vi "HFRR ADV v040.vi"() -> ()   [LabVIEW 2025] (continued)
          }
        }
        n1328 = case shown="True" w1638 {
          selector: w1638 -> [_ w1646]
          frame False {
          }
          frame True {
            n1329 = Not(x=w1646) -> (.not. x?=w1644:bool)
            n1330 = local write "CAMERA ROI MAX TEMP"(w1644) -> ()
            n1331 = call "IMAGE ANALYSIS.vi"("Enum"=POST_ANALYSIS_ENUM."SHOW UI") -> ("error out"=w1643:errorcluster)  [unwired: 9 in, 1 out]
            n1332 = call "LIST FILE NAMES.vi"("error in (no error)"=w1643) -> ("filenames"=w1642:string[])  [unwired: 9 in, 1 out]
            n1333 = property on="Test File List :" class="CmbBox"("Strings[]"=w1642) -> ()  [unwired: 2 in, 2 out]
          }
        }
        n1334 = local write "CAMERA ROI MIN TEMP"(TRUE ("CAMERA ROI MIN TEMP")) -> ()
      }
      frame "Compare Files" {
        n1335 = local read "LIVE FEED MIN TEMP"() -> (w1652:bool)
        n1336 = local write "LIVE FEED MAX TEMP"(TRUE ("LIVE FEED MAX TEMP")) -> ()
        n1337 = local read "CAMERA ROI MIN TEMP"() -> (w1650:bool)
        n1338 = case shown="True" w1652 {
          selector: w1652 -> [_ w1659]
          frame False {
          }
          frame True {
            n1339 = Not(x=w1659) -> (.not. x?=w1658:bool)
            n1340 = local write "LIVE FEED MIN TEMP"(w1658) -> ()
            n1341 = call "CAMERA LIVE FEED FGV.vi"("Enum - Menu"=CAMERA_LIVE_FEED_ENUM."CAMERA MINIMIZE") -> ()  [unwired: 9 in, 2 out]
          }
        }
        n1342 = case shown="True" w1650 {
          selector: w1650 -> [_ w1656]
          frame False {
          }
          frame True {
            n1343 = Not(x=w1656) -> (.not. x?=w1655:bool)
            n1344 = local write "CAMERA ROI MIN TEMP"(w1655) -> ()
            n1345 = call "IMAGE ANALYSIS.vi"("Enum"=POST_ANALYSIS_ENUM."MINIMIZE UI") -> ()  [unwired: 9 in, 2 out]
          }
        }
        n1346 = local write "CAMERA ROI MAX TEMP"(TRUE ("CAMERA ROI MAX TEMP")) -> ()
      }
      frame "About" {
        n1347 = local read "LIVE FEED MIN TEMP"() -> (w1662:bool)
        n1348 = local write "LIVE FEED MAX TEMP"(TRUE ("LIVE FEED MAX TEMP")) -> ()
        n1349 = local read "CAMERA ROI MIN TEMP"() -> (w1661:bool)
        n1350 = case shown="True" w1662 {
          selector: w1662 -> [_ w1669]
          frame False {
          }
          frame True {
            n1351 = Not(x=w1669) -> (.not. x?=w1668:bool)
            n1352 = local write "LIVE FEED MIN TEMP"(w1668) -> ()
            n1353 = call "CAMERA LIVE FEED FGV.vi"("Enum - Menu"=CAMERA_LIVE_FEED_ENUM."CAMERA MINIMIZE") -> ()  [unwired: 9 in, 2 out]
          }
        }
        n1354 = case shown="True" w1661 {
          selector: w1661 -> [_ w1666]
          frame False {
          }
          frame True {
            n1355 = Not(x=w1666) -> (.not. x?=w1665:bool)
            n1356 = local write "CAMERA ROI MIN TEMP"(w1665) -> ()
            n1357 = call "IMAGE ANALYSIS.vi"("Enum"=POST_ANALYSIS_ENUM."MINIMIZE UI") -> ()  [unwired: 9 in, 2 out]
          }
        }
        n1358 = local write "CAMERA ROI MAX TEMP"(TRUE ("CAMERA ROI MIN TEMP")) -> ()
      }
      frame "Advance" {
        n1359 = local read "LIVE FEED MIN TEMP"() -> (w1672:bool)
        n1360 = local write "LIVE FEED MAX TEMP"(TRUE ("LIVE FEED MAX TEMP")) -> ()
        n1361 = local read "CAMERA ROI MIN TEMP"() -> (w1670:bool)
        n1362 = case shown="True" w1672 {
          selector: w1672 -> [_ w1679]
          frame False {
          }
          frame True {
            n1363 = Not(x=w1679) -> (.not. x?=w1678:bool)
            n1364 = local write "LIVE FEED MIN TEMP"(w1678) -> ()
            n1365 = call "CAMERA LIVE FEED FGV.vi"("Enum - Menu"=CAMERA_LIVE_FEED_ENUM."CAMERA MINIMIZE") -> ()  [unwired: 9 in, 2 out]
          }
        }
        n1366 = local write "CAMERA ROI MAX TEMP"(TRUE ("CAMERA ROI MAX TEMP")) -> ()
        n1367 = case shown="True" w1670 {
          selector: w1670 -> [_ w1676]
          frame False {
          }
          frame True {
            n1368 = Not(x=w1676) -> (.not. x?=w1675:bool)
            n1369 = local write "CAMERA ROI MIN TEMP"(w1675) -> ()
            n1370 = call "IMAGE ANALYSIS.vi"("Enum"=POST_ANALYSIS_ENUM."MINIMIZE UI") -> ()  [unwired: 9 in, 2 out]
          }
        }
      }
      frame "Mooha" {
        n1371 = local read "LIVE FEED MIN TEMP"() -> (w1682:bool)
        n1372 = local write "LIVE FEED MAX TEMP"(TRUE ("LIVE FEED MAX TEMP")) -> ()
        n1373 = local read "CAMERA ROI MIN TEMP"() -> (w1680:bool)
        n1374 = case shown="True" w1682 {
          selector: w1682 -> [_ w1689]
          frame False {
          }
          frame True {
            n1375 = Not(x=w1689) -> (.not. x?=w1688:bool)
            n1376 = local write "LIVE FEED MIN TEMP"(w1688) -> ()
            n1377 = call "CAMERA LIVE FEED FGV.vi"("Enum - Menu"=CAMERA_LIVE_FEED_ENUM."CAMERA MINIMIZE") -> ()  [unwired: 9 in, 2 out]
          }
        }
        n1378 = local write "CAMERA ROI MAX TEMP"(TRUE ("CAMERA ROI MAX TEMP")) -> ()
        n1379 = case shown="True" w1680 {
          selector: w1680 -> [_ w1686]
          frame False {
          }
          frame True {
            n1380 = Not(x=w1686) -> (.not. x?=w1685:bool)
            n1381 = local write "CAMERA ROI MIN TEMP"(w1685) -> ()
            n1382 = call "IMAGE ANALYSIS.vi"("Enum"=POST_ANALYSIS_ENUM."MINIMIZE UI") -> ()  [unwired: 9 in, 2 out]
          }
        }
      }
    }
    n1383 = local read "Auto Start Test"() -> (w1427:bool)
    n1384 = case shown="True" "sign in temp" {
      frame False {
      }
      frame True {
        w1462 = 1 ("y")
        n1385 = local read "USERNAME"() -> (w1468:string)
        n1386 = local read "USER ID"() -> (w1465:string)
        n1387 = call <vilib>:"Trim Whitespace.vi"("string"=w1468) -> ("trimmed string"=w1467:string)  [unwired: 1 in]
        n1388 = call <vilib>:"Trim Whitespace.vi"("string"=w1465) -> ("trimmed string"=w1466:string)  [unwired: 1 in]
        n1389 = String Length(string=w1467) -> (length=w1464:i32)
        n1390 = String Length(string=w1466) -> (length=w1463:i32)
        n1391 = Greater?(x=w1464, y=w1462) -> (0:w1461:bool)
        n1392 = Greater?(x=w1463, y=w1462) -> (0:w1460:bool)
        n1393 = And(x=w1461, y=w1460) -> (x .and. y?=w1459:bool)
        n1394 = case shown="True" w1459 {
          frame False {
            n1395 = property on="Sign In" class="Bool (strict)"("DisabledEnum"=T19."Disabled" ("Disabled")) -> ()  [unwired: 2 in, 2 out]
          }
          frame True {
            n1396 = property on="Sign In" class="Bool (strict)"("DisabledEnum"=T19."Enabled" ("Disabled")) -> ()  [unwired: 2 in, 2 out]
          }
        }
      }
    }
    n1397 = local read "Air Temperature"() -> (w1444:bool)
    n1398 = local read "Coefficient Of Friction"() -> (w1445:bool)
    n1399 = case shown="False" w1427 {
      frame False {
        n1400 = local read "Auto stop temp"() -> (w1456:bool)
        n1401 = case shown="True" w1456 {
          frame False {
          }
          frame True {
            n1402 = local write "Auto Start Temp"(FALSE ("Auto Start Temp")) -> ()
          }
        }
      }
      frame True {
        "Auto stop temp" <- TRUE ("Auto stop temp")
      }
    }
    n1403 = local read "Humidity"() -> (w1443:bool)
    n1404 = case shown="\"HOME\"" w1453 {
      frame "HOME" {
        n1405 = local write "main tab sub"(enum32{"Page 1", "Page 2"}."Page 1" ("main tab sub")) -> ()
      }
      frame Default {
        n1406 = local write "main tab sub"(enum32{"Page 1", "Page 2"}."Page 2" ("main tab sub")) -> ()
      }
    }
    n1407 = case shown="True" w1452 {
      selector: w1452 -> [_ w1804]
      frame False {
      }
      frame True {
        n1408 = Not(x=w1804) -> (.not. x?=w1803:bool)
        n1409 = local write "Sign In"(w1803) -> ()
        n1410 = local write "Main Dashboard Buttons"(T26."Test Setup" ("Main Dashboard Buttons")) -> ()
      }
    }
    n1411 = case shown="\"Numeric Display\", Default" "Num/Graph" {
      frame "Numeric Display", Default {
        n1412 = property on="Single/Multiple" class="RadioBtnsControl (strict)"("Visible"=FALSE) -> ()  [unwired: 2 in, 2 out]
        n1413 = property on="Single - Graph" class="Ring (strict)"("Visible"=FALSE) -> ()  [unwired: 2 in, 2 out]
        n1414 = local write "Main Tab Display"(T4."Dashboard 1" ("Main Tab Display")) -> ()
      }
      frame "Graph Display" {
        n1415 = property on="Single/Multiple" class="RadioBtnsControl (strict)"("Visible"=TRUE) -> ()  [unwired: 2 in, 2 out]
        n1416 = case shown="\"Multiple\"" "Single/Multiple" {
          frame "Single ", Default {
            n1417 = property on="Single - Graph" class="Ring (strict)"("Visible"=TRUE) -> ()  [unwired: 2 in, 2 out]
            n1418 = local write "Main Tab Display"(T4."Dashboard 3" ("Main Tab Display")) -> ()
          }
          frame "Multiple" {
            n1419 = property on="Single - Graph" class="Ring (strict)"("Visible"=FALSE) -> ()  [unwired: 2 in, 2 out]
            n1420 = local write "Main Tab Display"(T4."Dashboard 2" ("Main Tab Display")) -> ()
          }
        }
      }
    }
    n1421 = local read "Stroke"() -> (w1442:bool)
    n1422 = local read "USERNAME"() -> (w1447:string)
    n1423 = case shown="True" w1445 {
      selector: w1445 -> [_ w1729]
      frame False {
      }
      frame True {
        n1424 = Not(x=w1729) -> (.not. x?=w1728:bool)
        n1425 = local write "Coefficient Of Friction"(w1728) -> ()
        n1426 = local write "Tab Control 2"(T6."Coefficient Of Friction" ("Tab Control 2")) -> ()
      }
    }
    n1427 = case shown="True" w1444 {
      selector: w1444 -> [_ w1726]
      frame False {
      }
      frame True {
        n1428 = Not(x=w1726) -> (.not. x?=w1724:bool)
        n1429 = local write "Air Temperature"(w1724) -> ()
        n1430 = local write "Tab Control 2"(T6."Air Temperature" ("Tab Control 2")) -> ()
      }
    }
    n1431 = case shown="True" w1442 {
      selector: w1442 -> [_ w1720]
      frame False {
      }
      frame True {
        n1432 = Not(x=w1720) -> (.not. x?=w1718:bool)
        n1433 = local write "Stroke"(w1718) -> ()
        n1434 = local write "Tab Control 2"(T6."Stroke" ("Tab Control 2")) -> ()
      }
    }
    n1435 = local write "tested by"(w1447) -> ()
    n1436 = case shown="True" w1443 {
      selector: w1443 -> [_ w1723]
      frame False {
      }
      frame True {
        n1437 = Not(x=w1723) -> (.not. x?=w1721:bool)
        n1438 = local write "Humidity"(w1721) -> ()
        n1439 = local write "Tab Control 2"(T6."Humidity" ("Tab Control 2")) -> ()
      }
    }
    n1440 = case shown="\"Calibration\"" "Main Dashboard Buttons" {
      tunnel: [T2."HOME" ("Main Tab") T2."Test Setup" ("Main Tab") T2."Acquire" ("Main Tab") T2."Adv Scar" ("Main Tab") T2."Adv Scar Report" ("Main Tab") T2."Compare Files" ("Main Tab") T2."Calibration" ("Main Tab") T2."About" ("Main Tab") T2."Advance" ("Main Tab")] -> w1426
      frame "Home", Default {
      }
      frame "Test Setup" {
      }
      frame "Dashboard" {
      }
      frame "Imaging" {
      }
      frame "Report" {
      }
      frame "Analysis" {
      }
      frame "Calibration" {
      }
      frame "About" {
      }
      frame "Advance" {
      }
    }
    n1441 = Wait (ms)(milliseconds to wait=u32 100) -> ()  [unwired: 1 out]
    n1442 = local read "Main Tab Display"() -> (w1446:T4)
    n1443 = local write "Main Tab"(w1426) -> ()
    n1444 = case shown="\"Dashboard 3\"" w1446 {
      frame "Dashboard 1", Default {
        n1445 = property on="Reset Graph" class="Bool (strict)"("Visible"=FALSE) -> ()  [unwired: 2 in, 2 out]
      }
      frame "Dashboard 2" {
        n1446 = property on="Reset Graph" class="Bool (strict)"("Visible"=TRUE) -> ()  [unwired: 2 in, 2 out]
      }
      frame "Dashboard 3" {
        n1447 = property on="Reset Graph" class="Bool (strict)"("Visible"=TRUE) -> ()  [unwired: 2 in, 2 out]
      }
    }
    n1448 = local read "SCAR MEASURMENT"() -> (w1434:enum32{"Auto Scar", "Manual Scar"})
    n1449 = local read "Humidity"() -> (w1448:bool)
    n1450 = local read "Cap Live Image"() -> (w1431:bool)
    n1451 = local read "Sample Temperature"() -> (w1441:bool)
    n1452 = local read "Air Temp vs Humidity"() -> (w1439:bool)
    n1453 = local read "Frequency"() -> (w1440:bool)
    n1454 = case shown="False" w1448 {
      frame False {
        n1455 = local write "Humidity On Command"(TRUE ("Humidity On Command")) -> ()
        n1456 = case shown="True" "Humidity Off Command" {
          selector: "Humidity Off Command" -> [_ w1736]
          frame False {
          }
          frame True {
            n1457 = stacked-sequence {
              frame #0 {
                n1458 = local read "WriteHumidity"() -> (w1738:string[])
                n1459 = Insert Into Array(array=w1738, new element="R;1" ("new element/subarray")) -> (w1737:string[])  [unwired: 1 in]
                n1460 = local write "WriteHumidity"(w1737) -> ()
              }
              frame #1 {
                n1461 = Wait (ms)(milliseconds to wait=u32 500) -> ()  [unwired: 1 out]
              }
              frame #2 {
                n1462 = local read "WriteHumidity"() -> (w1742:string[])
                n1463 = local read "EVENT LOG"() -> (w1746:string)
                n1464 = call "Event Log.vi"("Content"="Humidity Control Off" ("string"), "EVENT LOG"=w1746) -> ("EVENT LOG"=w1747:string)  [unwired: 8 in, 1 out]
                n1465 = local write "EVENT LOG"(w1747) -> ()
                n1466 = Insert Into Array(array=w1742, new element="R;1" ("new element/subarray")) -> (w1743:string[])  [unwired: 1 in]
                n1467 = local write "WriteHumidity"(w1743) -> ()
                n1468 = local write "Humidity 2"(TRUE ("Humidity")) -> ()
              }
            }
            n1469 = Not(x=w1736) -> (.not. x?=w1735:bool)
            n1470 = local write "Humidity Off Command"(w1735) -> ()
          }
        }
      }
      frame True {
        n1471 = local write "Humidity Off Command"(TRUE ("Humidity Off Command")) -> ()
        n1472 = case shown="False" "Humidity On Command" {
          selector: "Humidity On Command" -> [_ w1751]
          frame False {
          }
          frame True {
            n1473 = stacked-sequence {
              frame #0 {
                n1474 = local read "Set Rh"() -> (w1757:dbl)
                n1475 = local read "WriteHumidity"() -> (w1753:string[])
                n1476 = Number To Fractional String(number=w1757, precision (6)=i16 2) -> (F-format string=w1758:string)  [unwired: 2 in]
                n1477 = Concatenate Strings("M;" ("new element/subarray"), w1758) -> (w1756:string)
                n1478 = Insert Into Array(array=w1753, new element=w1756) -> (w1752:string[])  [unwired: 1 in]
                n1479 = local write "WriteHumidity"(w1752) -> ()
              }
              frame #1 {
                n1480 = Wait (ms)(milliseconds to wait=u32 500) -> ()  [unwired: 1 out]
              }
              frame #2 {
                n1481 = local read "WriteHumidity"() -> (w1761:string[])
                n1482 = local read "Set Rh"() -> (w1765:dbl)
                n1483 = Number To Fractional String(number=w1765, precision (6)=i16 2) -> (F-format string=w1766:string)  [unwired: 2 in]
                n1484 = Concatenate Strings("M;" ("new element/subarray"), w1766) -> (w1764:string)
                n1485 = Insert Into Array(array=w1761, new element=w1764) -> (w1760:string[])  [unwired: 1 in]
                n1486 = local write "WriteHumidity"(w1760) -> ()
              }
              frame #3 {
                n1487 = Wait (ms)(milliseconds to wait=u32 500) -> ()  [unwired: 1 out]
              }
              frame #4 {
                (unwired) "% RH" ("string")
                (unwired) i16 2 ("precision (6)")
                (unwired) "M;" ("new element/subarray")
                n1488 = local read "Set Rh"() -> (w1775:dbl)
                n1489 = local read "WriteHumidity"() -> (w1768:string[])
                n1490 = Number To Fractional String(number=w1775, precision (6)=i16 2) -> (F-format string=w1772:string)  [unwired: 2 in]
                n1491 = Concatenate Strings("M;" ("new element/subarray"), w1772) -> (w1776:string)
                n1492 = Concatenate Strings("Humidity Set to : " ("string"), w1772, "% RH" ("string")) -> (w1770:string)
                n1493 = Insert Into Array(array=w1768, new element=w1776) -> (w1769:string[])  [unwired: 1 in]
                n1494 = disable-structure shown="Enabled" {
                  frame Enabled {
                    n1495 = local read "EVENT LOG"() -> (w1779:string)
                    n1496 = call "Event Log.vi"("Content"="Humidity Control On", "EVENT LOG"=w1779) -> ("EVENT LOG"=w1780:string)  [unwired: 8 in, 1 out]
                    n1497 = local write "EVENT LOG"(w1780) -> ()
                  }
                  frame Disabled {
                  }
                }
                n1498 = disable-structure shown="Enabled" {
                  disable-tunnel: w1770 -> [_ _]
                  frame Enabled {
                    n1499 = local read "EVENT LOG"() -> (w1782:string)
                    n1500 = call "Event Log.vi"("Content"="Humidity Control On", "EVENT LOG"=w1782) -> ("EVENT LOG"=w1783:string)  [unwired: 8 in, 1 out]
                    n1501 = local write "EVENT LOG"(w1783) -> ()
                  }
                  frame Disabled {
                  }
                }
                n1502 = local write "WriteHumidity"(w1769) -> ()
              }
            }
            n1503 = Not(x=w1751) -> (.not. x?=w1750:bool)
            n1504 = local write "Humidity On Command"(w1750) -> ()
          }
        }
      }
    }
    n1505 = Equal?(x=w1434, y=enum32{"Auto Scar", "Manual Scar"}."Auto Scar" ("SCAR MEASURMENT")) -> (x = y?=w1430:bool)
    n1506 = local read "TEST STANDARD"() -> (w1437:T3)
    n1507 = And(x=w1431, y=w1430) -> (x .and. y?=w1432:bool)
    n1508 = case shown="True" w1432 {
      selector: w1432 -> [_ w1535]
      tunnel: errorcluster {"status"=FALSE, "code"=0, "source"=""} ("error in (no error) 3") -> [_ w1536]
      frame False {
      }
      frame True {
        n1509 = stacked-sequence {
          tunnel: w1536 -> [_ _ _ _ _ _ _ w1584]
          tunnel: w1535 -> [_ _ _ _ _ w1565 _ _]
          frame #0 {
            n1510 = call "CAMERA LIVE FEED FGV.vi"("Enum - Menu"=CAMERA_LIVE_FEED_ENUM."CAMERA MINIMIZE") -> ()  [unwired: 9 in, 2 out]
          }
          frame #1 {
            n1511 = property on="Auto Scar Check  2" class="Clust (strict)"("Visible"=TRUE) -> ()  [unwired: 2 in, 2 out]
          }
          frame #2 {
            n1512 = String To Path(string="C:\\LAB-IQ\\Image Calibrate v01.dcf") -> (path=w1541:path)
            n1513 = Open/Create/Replace File ("Open File")(file path (use dialog)=w1541) -> (refnum out=w1542:refnum<file>)  [unwired: 5 in, 2 out]
            n1514 = for {
              N: 4 -> [_]
              tunnel: w1542 -> [w1548]
              i -> [w1544]
              n1515 = Read from Text File ("Read File")(file (use dialog)=w1548) -> (text=w1549:string)  [unwired: 3 in, 3 out]
              n1516 = String Subset(string=w1549, offset (0)=6, length (rest)=10 ("length (rest)")) -> (substring=w1545:string)
              n1517 = Fract/Exp String To Number(string=w1545) -> (number=w1543:dbl)  [unwired: 3 in, 1 out]
              n1518 = case shown="0" w1544 {
                tunnel: w1543 -> [w1550 w1551 _ w1552 _]
                frame 0 {
                  "5x Gain" <- w1550
                }
                frame 1 {
                  "10x Gain" <- w1551
                }
                frame 2 {
                }
                frame 3 {
                  "100x gain" <- w1552
                }
                frame 4, Default {
                }
              }
            }
          }
          frame #3 {
            n1519 = local read "FILE 3"() -> (w1558:string)
            n1520 = call <vilib>:"Trim Whitespace.vi"("string"="C:\\LAB-IQ\\images\\") -> ("trimmed string"=w1560:string)  [unwired: 1 in]
            n1521 = String To Path(string=w1560) -> (path=w1559:path)
            n1522 = Concatenate Strings(w1558, ".png" ("string")) -> (w1557:string)
            n1523 = Build Path(base path=w1559, name or relative path=w1557) -> (appended path=w1555:path)
            "Image path" <- w1555
            n1524 = Path To String(path=w1555) -> (string=w1554:string)
            n1525 = call "CAMERA LIVE FEED FGV.vi"("Enum - Menu"=CAMERA_LIVE_FEED_ENUM."CAMERA SAVE", "Image Path"=w1554) -> ()  [unwired: 8 in, 2 out]
          }
          frame #4 {
            n1526 = One Button Dialog(message="Image saved successfully") -> ()  [unwired: 1 in, 1 out]
          }
          frame #5 {
            n1527 = local read "TEST STANDARD"() -> (w1564:T3)
            n1528 = local read "Magnification len live scar"() -> (w1576:string)
            n1529 = Not(x=w1565) -> (.not. x?=w1566:bool)
            n1530 = local write "Cap Live Image"(w1566) -> ()
            n1531 = case shown="\"ISO 12156\"" w1564 {
              tunnel: ["ASTM D6079" "ISO 12156"] -> w1563
              frame "ASTM D6079", Default {
              }
              frame "ISO 12156" {
              }
            }
            n1532 = case shown="\"5x\", Default" w1576 {
              tunnel: [w1579 w1580] -> w1575
              frame "5x", Default {
                n1533 = local read "5x Gain"() -> (w1579:dbl)
              }
              frame "10x" {
                # "5x"
                n1534 = local read "10x Gain"() -> (w1580:dbl)
              }
            }
            n1535 = local read "Image path"() -> (w1574:path)
            n1536 = local read "FILE 3"() -> (w1567:string)
            n1537 = call "EDGE DETCTION.vi"("GAIN VALUE"=w1575, "Image Path"=w1574) -> ("error out"=w1573:errorcluster, "return value"=w1572:cluster{string, string, dbl, dbl, dbl})  [unwired: 8 in]
            n1538 = Bundle By Name(cluster=T27 {"File Name"="", "Test Method"="", "Operator"="", "Fuel Description"="", "Date and time"=""} ("Main Ref"), "File Name"=w1567, "Test Method"=w1563) -> (w1568:T27)
            n1539 = call "duf file read.vi"("error in (no error)"=w1573, "Main Ref"=w1568) -> ("error out"=w1571:errorcluster, "Main Ref 2"=w1569:T27)  [unwired: 8 in]
            n1540 = call "EDGE DETECTION REPORT.vi"("error in (no error)"=w1571, "return value 2"=w1572, "Main Ref"=w1569) -> ()  [unwired: 8 in, 1 out]
          }
          frame #6 {
            n1541 = property on="Auto Scar Check  2" class="Clust (strict)"("Visible"=FALSE) -> ()  [unwired: 2 in, 2 out]
          }
          frame #7 {
            n1542 = call "CAMERA LIVE FEED FGV.vi"("Enum - Menu"=CAMERA_LIVE_FEED_ENUM."CAMERA MINIMIZE", "error in (no error)"=w1584) -> ()  [unwired: 8 in, 2 out]
            n1543 = local write "Main Dashboard Buttons"(T1."Home" ("Main Dashboard Buttons")) -> ()
            n1544 = local write "Main Tab"(T2."HOME" ("Main Tab")) -> ()
          }
        }
      }
    }
    n1545 = local read "Heater Button"() -> (w1438:bool)
    n1546 = case shown="True" w1440 {
      selector: w1440 -> [_ w1714]
      frame False {
      }
      frame True {
        n1547 = Not(x=w1714) -> (.not. x?=w1712:bool)
        n1548 = local write "Frequency"(w1712) -> ()
        n1549 = local write "Tab Control 2"(T6."Frequency" ("Tab Control 2")) -> ()
      }
    }
    n1550 = case shown="True" w1439 {
      selector: w1439 -> [_ w1711]
      frame False {
      }
      frame True {
        n1551 = Not(x=w1711) -> (.not. x?=w1709:bool)
        n1552 = local write "Air Temp vs Humidity"(w1709) -> ()
        n1553 = local write "Tab Control 2"(T6."Air Temp vs Rh" ("Tab Control 2")) -> ()
      }
    }
    n1554 = case shown="True" w1441 {
      selector: w1441 -> [_ w1717]
      frame False {
      }
      frame True {
        n1555 = Not(x=w1717) -> (.not. x?=w1715:bool)
        n1556 = local write "Sample Temperature"(w1715) -> ()
        n1557 = local write "Tab Control 2"(T6."Sample Temperature" ("Tab Control 2")) -> ()
      }
    }
    n1558 = case shown="\"Custom\"" w1437 {
      frame "ASTM D6079", Default {
        w1690 = "ASTM D6079 TEST CONDITIONS" ("Standard 2")
        n1559 = local write "Standard 2"(w1690) -> ()
        n1560 = local write "Standard"(w1690) -> ()
      }
      frame "ISO 12156" {
        w1691 = "ISO 12156 TEST CONDITIONS" ("Standard 2")
        n1561 = local write "Standard 2"(w1691) -> ()
        n1562 = local write "Standard"(w1691) -> ()
      }
      frame "CEC F-096-A-06" {
        w1692 = "CEC F-096-A-06 TEST CONDITIONS" ("Standard 2")
        n1563 = local write "Standard 2"(w1692) -> ()
        n1564 = local write "Standard"(w1692) -> ()
      }
      frame "Custom" {
        w1693 = "CUSTOM TEST CONDITIONS" ("Standard 2")
        n1565 = local write "Standard 2"(w1693) -> ()
        n1566 = local write "Standard"(w1693) -> ()
      }
    }
    n1567 = case shown="True" w1438 {
      frame False {
        n1568 = local write "Temperature On Command"(TRUE ("Temperature On Command")) -> ()
        n1569 = case shown="True" "Temperature Off Command" {
          selector: "Temperature Off Command" -> [_ w1697]
          frame False {
          }
          frame True {
            n1570 = Not(x=w1697) -> (.not. x?=w1696:bool)
            n1571 = local read "EVENT LOG"() -> (w1700:string)
            n1572 = local write "Temperature Off Command"(w1696) -> ()
            n1573 = call "Event Log.vi"("Content"="Heater Off", "EVENT LOG"=w1700) -> ("EVENT LOG"=w1699:string)  [unwired: 8 in, 1 out]
            n1574 = local write "EVENT LOG"(w1699) -> ()
          }
        }
      }
      frame True {
        n1575 = local write "Temperature Off Command"(TRUE ("Temperature Off Command")) -> ()
        n1576 = case shown="True" "Temperature On Command" {
          selector: "Temperature On Command" -> [_ w1704]
          frame False {
          }
          frame True {
            n1577 = Not(x=w1704) -> (.not. x?=w1703:bool)
            n1578 = local write "Temperature On Command"(w1703) -> ()
            n1579 = disable-structure shown="Enabled" {
              disable-tunnel: "Heater On" -> [w1706 _]
              frame Enabled {
                n1580 = local read "EVENT LOG"() -> (w1707:string)
                n1581 = call "Event Log.vi"("Content"=w1706, "EVENT LOG"=w1707) -> ("EVENT LOG"=w1708:string)  [unwired: 8 in, 1 out]
                n1582 = local write "EVENT LOG"(w1708) -> ()
              }
              frame Disabled {
              }
            }
          }
        }
      }
    }
    n1583 = local read "Main Tab"() -> (w1429:T2)
    n1584 = case shown="\"About\"" w1429 {
      frame "HOME", Default {
        w1471 = T19."Enabled" ("Disabled")
        n1585 = local read "Service Password enable"() -> (w1473:bool)
        n1586 = property on="Imaging" class="Bool (strict)"("DisabledEnum"=w1471) -> ()  [unwired: 2 in, 2 out]
        n1587 = property on="Dashboard" class="Bool (strict)"("DisabledEnum"=w1471) -> ()  [unwired: 2 in, 2 out]
        n1588 = property on="Test Setup" class="Bool (strict)"("DisabledEnum"=w1471) -> ()  [unwired: 2 in, 2 out]
        n1589 = property on="Analysis" class="Bool (strict)"("DisabledEnum"=w1471) -> ()  [unwired: 2 in, 2 out]
        n1590 = property on="Home" class="Bool (strict)"("DisabledEnum"=w1471) -> ()  [unwired: 2 in, 2 out]
        n1591 = property on="Report" class="Bool (strict)"("DisabledEnum"=w1471) -> ()  [unwired: 2 in, 2 out]
        n1592 = property on="Main Dashboard Buttons" class="RadioBtnsControl (strict)"("DisabledEnum"=w1471) -> ()  [unwired: 2 in, 2 out]
        n1593 = property on="Calibration" class="Bool (strict)"("DisabledEnum"=w1471) -> ()  [unwired: 2 in, 2 out]
        n1594 = case shown="True" w1473 {
          tunnel: [T19."Disabled" ("Disabled") T19."Enabled" ("Disabled")] -> w1472
          frame False {
          }
          frame True {
          }
        }
        n1595 = property on="About" class="Bool (strict)"("DisabledEnum"=w1472) -> ()  [unwired: 2 in, 2 out]
      }
      frame "Test Setup" {
        w1478 = T19."Enabled" ("Disabled")
        n1596 = local read "Service Password enable"() -> (w1477:bool)
        n1597 = property on="Dashboard" class="Bool (strict)"("DisabledEnum"=T19."Disabled" ("Disabled")) -> ()  [unwired: 2 in, 2 out]
        n1598 = property on="Imaging" class="Bool (strict)"("DisabledEnum"=w1478) -> ()  [unwired: 2 in, 2 out]
        n1599 = property on="Analysis" class="Bool (strict)"("DisabledEnum"=w1478) -> ()  [unwired: 2 in, 2 out]
        n1600 = property on="Home" class="Bool (strict)"("DisabledEnum"=w1478) -> ()  [unwired: 2 in, 2 out]
        n1601 = property on="Report" class="Bool (strict)"("DisabledEnum"=w1478) -> ()  [unwired: 2 in, 2 out]
        n1602 = property on="Test Setup" class="Bool (strict)"("DisabledEnum"=w1478) -> ()  [unwired: 2 in, 2 out]
        n1603 = case shown="True" w1477 {
          tunnel: [T19."Disabled" ("Disabled") T19."Enabled" ("Disabled")] -> w1476
          frame False {
          }
          frame True {
          }
        }
        n1604 = property on="About" class="Bool (strict)"("DisabledEnum"=w1476) -> ()  [unwired: 2 in, 2 out]
      }
      frame "Adv Scar" {
        w1485 = T19."Enabled" ("Disabled")
        n1605 = property on="Dashboard" class="Bool (strict)"("DisabledEnum"=T19."Disabled" ("Disabled")) -> ()  [unwired: 2 in, 2 out]
        n1606 = property on="Imaging" class="Bool (strict)"("DisabledEnum"=w1485) -> ()  [unwired: 2 in, 2 out]
        n1607 = property on="Analysis" class="Bool (strict)"("DisabledEnum"=w1485) -> ()  [unwired: 2 in, 2 out]
        n1608 = property on="Home" class="Bool (strict)"("DisabledEnum"=w1485) -> ()  [unwired: 2 in, 2 out]
        n1609 = property on="Report" class="Bool (strict)"("DisabledEnum"=w1485) -> ()  [unwired: 2 in, 2 out]
        n1610 = property on="Test Setup" class="Bool (strict)"("DisabledEnum"=w1485) -> ()  [unwired: 2 in, 2 out]
        n1611 = local read "Service Password enable"() -> (w1483:bool)
        n1612 = case shown="True" w1483 {
          tunnel: [T19."Disabled" ("Disabled") T19."Enabled" ("Disabled")] -> w1482
          frame False {
          }
          frame True {
          }
        }
        n1613 = property on="About" class="Bool (strict)"("DisabledEnum"=w1482) -> ()  [unwired: 2 in, 2 out]
      }
      frame "Calibration" {
        w1488 = T19."Enabled" ("Disabled")
        n1614 = property on="Dashboard" class="Bool (strict)"("DisabledEnum"=T19."Disabled" ("Disabled")) -> ()  [unwired: 2 in, 2 out]
        n1615 = property on="Imaging" class="Bool (strict)"("DisabledEnum"=w1488) -> ()  [unwired: 2 in, 2 out]
        n1616 = property on="Analysis" class="Bool (strict)"("DisabledEnum"=w1488) -> ()  [unwired: 2 in, 2 out]
        n1617 = property on="Home" class="Bool (strict)"("DisabledEnum"=w1488) -> ()  [unwired: 2 in, 2 out]
        n1618 = property on="Report" class="Bool (strict)"("DisabledEnum"=w1488) -> ()  [unwired: 2 in, 2 out]
        n1619 = property on="Test Setup" class="Bool (strict)"("DisabledEnum"=w1488) -> ()  [unwired: 2 in, 2 out]
        n1620 = local read "Service Password enable"() -> (w1490:bool)
        n1621 = property on="Calibration" class="Bool (strict)"("DisabledEnum"=w1488) -> ()  [unwired: 2 in, 2 out]
        n1622 = case shown="True" w1490 {
          tunnel: [T19."Disabled" ("Disabled") T19."Enabled" ("Disabled")] -> w1489
          frame False {
          }
          frame True {
          }
        }
        n1623 = property on="About" class="Bool (strict)"("DisabledEnum"=w1489) -> ()  [unwired: 2 in, 2 out]
      }
      frame "Adv Scar Report" {
        w1496 = T19."Enabled" ("Disabled")
        n1624 = property on="Dashboard" class="Bool (strict)"("DisabledEnum"=T19."Disabled" ("Disabled")) -> ()  [unwired: 2 in, 2 out]
        n1625 = property on="Imaging" class="Bool (strict)"("DisabledEnum"=w1496) -> ()  [unwired: 2 in, 2 out]
        n1626 = property on="Analysis" class="Bool (strict)"("DisabledEnum"=w1496) -> ()  [unwired: 2 in, 2 out]
        n1627 = property on="Home" class="Bool (strict)"("DisabledEnum"=w1496) -> ()  [unwired: 2 in, 2 out]
        n1628 = property on="Report" class="Bool (strict)"("DisabledEnum"=w1496) -> ()  [unwired: 2 in, 2 out]
        n1629 = property on="Test Setup" class="Bool (strict)"("DisabledEnum"=w1496) -> ()  [unwired: 2 in, 2 out]
        n1630 = local read "Service Password enable"() -> (w1495:bool)
        n1631 = case shown="True" w1495 {
          tunnel: [T19."Disabled" ("Disabled") T19."Enabled" ("Disabled")] -> w1494
          frame False {
          }
          frame True {
          }
        }
        n1632 = property on="About" class="Bool (strict)"("DisabledEnum"=w1494) -> ()  [unwired: 2 in, 2 out]
      }
      frame "Compare Files" {
        w1502 = T19."Enabled" ("Disabled")
        n1633 = local read "Service Password enable"() -> (w1501:bool)
        n1634 = property on="Dashboard" class="Bool (strict)"("DisabledEnum"=T19."Disabled" ("Disabled")) -> ()  [unwired: 2 in, 2 out]
        n1635 = property on="Imaging" class="Bool (strict)"("DisabledEnum"=w1502) -> ()  [unwired: 2 in, 2 out]
        n1636 = property on="Analysis" class="Bool (strict)"("DisabledEnum"=w1502) -> ()  [unwired: 2 in, 2 out]
        n1637 = property on="Home" class="Bool (strict)"("DisabledEnum"=w1502) -> ()  [unwired: 2 in, 2 out]
        n1638 = property on="Report" class="Bool (strict)"("DisabledEnum"=w1502) -> ()  [unwired: 2 in, 2 out]
        n1639 = property on="Test Setup" class="Bool (strict)"("DisabledEnum"=w1502) -> ()  [unwired: 2 in, 2 out]
        n1640 = case shown="True" w1501 {
          tunnel: [T19."Disabled" ("Disabled") T19."Enabled" ("Disabled")] -> w1500
          frame False {
          }
          frame True {
          }
        }
        n1641 = property on="About" class="Bool (strict)"("DisabledEnum"=w1500) -> ()  [unwired: 2 in, 2 out]
      }
      frame "Acquire" {
        n1642 = local read "Service Password enable"() -> (w1507:bool)
        n1643 = property on="Test Setup" class="Bool (strict)"("DisabledEnum"=T19."Disabled" ("Disabled")) -> ()  [unwired: 2 in, 2 out]
        n1644 = local read "Auto Start Test"() -> (w1509:bool)
        n1645 = local read "RUN"() -> (w1511:bool)
        n1646 = case shown="True" w1507 {
          tunnel: [T19."Disabled" ("Disabled") T19."Enabled" ("Disabled")] -> w1508
          frame False {
          }
          frame True {
          }
        }
        n1647 = Or(x=w1511, y=w1509) -> (x .or. y?=w1510:bool)
        n1648 = case shown="True" w1510 {
          tunnel: [T19."Enabled" ("Disabled") T19."Disabled" ("Disabled")] -> w1506
          frame False {
          }
          frame True {
          }
        }
        n1649 = property on="About" class="Bool (strict)"("DisabledEnum"=w1508) -> ()  [unwired: 2 in, 2 out]
        n1650 = property on="Imaging" class="Bool (strict)"("DisabledEnum"=w1506) -> ()  [unwired: 2 in, 2 out]
        n1651 = property on="Dashboard" class="Bool (strict)"("DisabledEnum"=w1506) -> ()  [unwired: 2 in, 2 out]
        n1652 = property on="Analysis" class="Bool (strict)"("DisabledEnum"=w1506) -> ()  [unwired: 2 in, 2 out]
        n1653 = property on="Home" class="Bool (strict)"("DisabledEnum"=w1506) -> ()  [unwired: 2 in, 2 out]
        n1654 = property on="Report" class="Bool (strict)"("DisabledEnum"=w1506) -> ()  [unwired: 2 in, 2 out]
        n1655 = property on="Calibration" class="Bool (strict)"("DisabledEnum"=w1506) -> ()  [unwired: 2 in, 2 out]
      }
      frame "About" {
        n1656 = local read "FILE"() -> (w1525:string)
        n1657 = local read "TEST FILE NAM,E SAVED"() -> (w1518:bool)
        n1658 = call <vilib>:"Trim Whitespace.vi"("string"=w1525) -> ("trimmed string"=w1524:string)  [unwired: 1 in]
        n1659 = local read "Auto Start Test"() -> (w1528:bool)
        n1660 = String Length(string=w1524) -> (length=w1523:i32)
        n1661 = Greater?(x=w1523, y=1) -> (0:w1520:bool)
        n1662 = And(x=w1520, y=w1518) -> (x .and. y?=w1519:bool)
        n1663 = local read "RUN"() -> (w1530:bool)
        n1664 = case shown="True" w1519 {
          tunnel: [T19."Disabled" ("Disabled") T19."Enabled" ("Disabled")] -> w1521
          frame False {
          }
          frame True {
          }
        }
        n1665 = Or(x=w1530, y=w1528) -> (x .or. y?=w1529:bool)
        n1666 = property on="About" class="Bool (strict)"("DisabledEnum"=T19."Enabled" ("Disabled")) -> ()  [unwired: 2 in, 2 out]
        n1667 = case shown="False" w1529 {
          tunnel: [T19."Enabled" ("Disabled") T19."Disabled" ("Disabled")] -> w1527
          frame False {
          }
          frame True {
          }
        }
        n1668 = property on="Dashboard" class="Bool (strict)"("DisabledEnum"=w1521) -> ()  [unwired: 2 in, 2 out]
        n1669 = property on="Test Setup" class="Bool (strict)"("DisabledEnum"=T19."Disabled" ("Disabled")) -> ()  [unwired: 2 in, 2 out]
        n1670 = property on="Imaging" class="Bool (strict)"("DisabledEnum"=w1527) -> ()  [unwired: 2 in, 2 out]
        n1671 = property on="Analysis" class="Bool (strict)"("DisabledEnum"=w1527) -> ()  [unwired: 2 in, 2 out]
        n1672 = property on="Home" class="Bool (strict)"("DisabledEnum"=w1527) -> ()  [unwired: 2 in, 2 out]
        n1673 = property on="Report" class="Bool (strict)"("DisabledEnum"=w1527) -> ()  [unwired: 2 in, 2 out]
      }
    }
    n1674 = local read "Quit"() -> (w1455:bool)
    "Single" <- "Single - Graph"
  }
  n1675 = disable-structure shown="Disabled" {
    disable-tunnel: [w1808 _] -> w44
    disable-tunnel: _ -> [w1807 _]
    frame Disabled {
      n1676 = while {
        tunnel: w1807 -> [_]
        tunnel: [w1809] -> w1808
        tunnel: [w1810] -> _
        i -> [w1810]
        stop <- w1809 stop-if-true
        w1826 = u16 10 items=["1.0"=10, "1.5"=15, "2.0"=20] ("stop bits (10: 1 bit)")
        n1677 = Wait (ms)(milliseconds to wait=u32 10) -> ()  [unwired: 1 out]
        n1678 = call-poly "VISA Configure Serial Port"("VISA resource name"=refnum<visa-resource-name> "ASRL1::INSTR" ("COM PORT"), "timeout (10sec)"=u32 10, "baud rate (9600)"=u32 57600, "data bits (8)"=u16 8, "stop bits (10: 1 bit)"=w1826) -> ("VISA resource name out"=w1812:refnum<visa-resource-name>, "error out"=w1821:errorcluster)  [unwired: 9 in]
        n1679 = VISA Read(VISA resource name=w1812, byte count=u32 2 ("byte count (0)")) -> (read buffer=w1820:string)  [unwired: 1 in, 3 out]
        n1680 = String Subset(string=w1820, offset (0)=0, length (rest)=2 ("length (rest)")) -> (substring=w1819:string)
        n1681 = Match Pattern(string=w1819, regular expression="<>") -> (offset past match=w1816:i32)  [unwired: 1 in, 3 out]
        n1682 = Greater Or Equal?(x=w1816, y=0) -> (x >= y?=w1811:bool)
        n1683 = case shown="True" w1811 {
          tunnel: w1812 -> [_ w1830]
          tunnel: w1821 -> [_ w1829]
          frame False {
          }
          frame True {
            n1684 = VISA Read(VISA resource name=w1830, byte count=u32 32 ("byte count (0)"), error in (no error)=w1829) -> (read buffer=w1828:string)  [unwired: 3 out]
            n1685 = String Subset(string=w1828, offset (0)=0, length (rest)=8 ("length (rest)")) -> (substring=w1832:string)
            n1686 = String Subset(string=w1828, offset (0)=8, length (rest)=8 ("length (rest)")) -> (substring=w1833:string)
            n1687 = Decimal String To Number(string=w1833) -> (number=w1840:i32)  [unwired: 2 in, 1 out]
            n1688 = Decimal String To Number(string=w1832) -> (number=w1836:i32)  [unwired: 2 in, 1 out]
            n1689 = Divide(x=w1840, y=10000) -> ()  [unwired: 1 out]
            n1690 = Divide(x=w1836, y=1000000) -> ()  [unwired: 1 out]
          }
        }
        n1691 = local read "Quit"() -> (w1809:bool)
      }
    }
    frame Enabled {
    }
  }
  n1692 = Tick Count (ms)() -> (millisecond timer value=w6:u32)
  n1693 = while {
    shift-right: [w1886] -> _
    shift-left: w8 -> [w1890]
    shift-right: [w1885] -> _
    shift-left: w7 -> [w1889]
    shift-right: [w1884] -> _
    shift-left: w8 -> [w1888]
    shift-right: [w1883] -> _
    shift-left: w7 -> [w1887]
    shift-right: [w1881] -> _
    shift-left: w6 -> [w1882]
    shift-right: [w1878] -> _
    shift-left: w5 -> [w1879]
    shift-right: [w1877] -> _
    shift-left: w5 -> [w1880]
    shift-right: [w1870] -> _
    shift-left: w5 -> [w1876]
    shift-right: [w1869] -> _
    shift-left: w5 -> [w1875]
    shift-right: [w1868] -> _
    shift-left: w5 -> [w1874]
    shift-right: [w1867] -> _
    shift-left: w5 -> [w1873]
    shift-right: [w1866] -> _
    shift-left: w5 -> [w1872]
    shift-right: [w1865] -> _
    shift-left: w5 -> [w1871]
    shift-right: [w1864] -> _
    shift-left: w5 -> [w1858]
    shift-right: [w1863] -> _
    shift-left: w5 -> [w1857]
    shift-right: [w1862] -> _
    shift-left: w5 -> [w1856]
    shift-right: [w1861] -> _
    shift-left: w5 -> [w1855]
    shift-right: [w1860] -> _
    shift-left: w5 -> [w1854]
    shift-right: [w1859] -> _
    shift-left: w5 -> [w1853]
    shift-right: [w1844] -> _
    shift-left: w5 -> [w1847]
    shift-right: [w1843] -> _
    shift-left: w5 -> [w1846]
    shift-right: [w1842] -> _
    shift-left: w5 -> [w1845]
    stop <- w1892 stop-if-true
    n1694 = local read "Read UNO"() -> (w1851:string)
    n1695 = local read "Error  2"() -> (w1891:errorcluster)
    n1696 = String Length(string=w1851) -> (length=w1850:i32)
    n1697 = call <vilib>:"Trim Whitespace.vi"("string"=w1851) -> ("trimmed string"=w1852:string)  [unwired: 1 in]
    n1698 = Greater Or Equal?(x=w1850, y=23) -> (x >= y?=w1848:bool)
    n1699 = case shown="No Error" w1891 {
      tunnel: w1890 -> [w1938 w2034]
      tunnel: w1889 -> [w1937 w2033]
      tunnel: w1888 -> [w1936 w2032]
      tunnel: w1887 -> [w1935 w2031]
      tunnel: [w1934 w2034] -> w1886
      tunnel: [w1933 w2033] -> w1885
      tunnel: [w1932 w2032] -> w1884
      tunnel: [w1931 w2031] -> w1883
      tunnel: w1882 -> [w1930 w2030]
      tunnel: [w1929 w2030] -> w1881
      tunnel: w1879 -> [w1928 w2029]
      tunnel: w1880 -> [w1927 w2028]
      tunnel: [w1926 w2029] -> w1878
      tunnel: [w1925 w2028] -> w1877
      tunnel: w1876 -> [w1924 w2027]
      tunnel: w1875 -> [w1923 w2026]
      tunnel: w1874 -> [w1922 w2025]
      tunnel: w1873 -> [w1921 w2024]
      tunnel: w1872 -> [w1920 w2023]
      tunnel: w1871 -> [w1919 w2022]
      tunnel: [w1918 w2027] -> w1870
      tunnel: [w1917 w2026] -> w1869
      tunnel: [w1916 w2025] -> w1868
      tunnel: [w1915 w2024] -> w1867
      tunnel: [w1914 w2023] -> w1866
      tunnel: [w1913 w2022] -> w1865
      tunnel: w1858 -> [w1912 w2021]
      tunnel: [w1911 w2021] -> w1864
      tunnel: [w1910 w2017] -> w1863
      tunnel: [w1909 w2016] -> w1862
      tunnel: [w1908 w2020] -> w1861
      tunnel: [w1907 w2019] -> w1860
      tunnel: [w1906 w2018] -> w1859
      tunnel: w1857 -> [w1905 w2020]
      tunnel: w1856 -> [w1904 w2019]
      tunnel: w1855 -> [w1903 w2018]
      tunnel: w1854 -> [w1902 w2017]
      tunnel: w1853 -> [w1901 w2016]
      tunnel: w1852 -> [w1900 _]
      tunnel: w1848 -> [w1899 _]
      tunnel: w1847 -> [w1898 w2015]
      tunnel: w1846 -> [w1897 w2014]
      tunnel: w1845 -> [w1896 w2013]
      tunnel: [w1895 w2015] -> w1844
      tunnel: [w1894 w2014] -> w1843
      tunnel: [w1893 w2013] -> w1842
      frame No Error {
        n1700 = case shown="True" w1899 {
          tunnel: w1938 -> [w1954 w2006]
          tunnel: w1937 -> [w1953 w2005]
          tunnel: w1936 -> [w1952 w2004]
          tunnel: w1935 -> [w1951 w2003]
          tunnel: [w1954 w2002] -> w1934
          tunnel: [w1953 w2001] -> w1933
          tunnel: [w1952 w2000] -> w1932
          tunnel: [w1951 w1999] -> w1931
          tunnel: w1930 -> [w1950 w1997]
          tunnel: [w1950 w1996] -> w1929
          tunnel: w1928 -> [w1949 w1995]
          tunnel: w1927 -> [w1948 w1994]
          tunnel: [w1949 w1993] -> w1926
          tunnel: [w1948 w1992] -> w1925
          tunnel: w1924 -> [w1947 w1991]
          tunnel: w1923 -> [w1946 w1990]
          tunnel: w1922 -> [w1945 w1989]
          tunnel: w1921 -> [w1944 w1988]
          tunnel: w1920 -> [w1943 w1987]
          tunnel: w1919 -> [w1942 w1986]
          tunnel: [w1947 w1985] -> w1918
          tunnel: [w1946 w1984] -> w1917
          tunnel: [w1945 w1983] -> w1916
          tunnel: [w1944 w1982] -> w1915
          tunnel: [w1943 w1981] -> w1914
          tunnel: [w1942 w1980] -> w1913
          tunnel: w1912 -> [w1960 w1979]
          tunnel: [w1960 w1978] -> w1911
          tunnel: [w1957 w1977] -> w1910
          tunnel: [w1956 w1976] -> w1909
          tunnel: [w1959 w1975] -> w1908
          tunnel: [w1955 w1974] -> w1907
          tunnel: [w1958 w1973] -> w1906
          tunnel: w1905 -> [w1959 w1972]
          tunnel: w1904 -> [w1958 w1971]
          tunnel: w1903 -> [w1957 w1970]
          tunnel: w1902 -> [w1956 w1969]
          tunnel: w1901 -> [w1955 w1968]
          tunnel: w1900 -> [_ w1967]
          tunnel: w1898 -> [w1941 w1966]
          tunnel: w1897 -> [w1940 w1965]
          tunnel: w1896 -> [w1939 w1964]
          tunnel: [w1941 w1963] -> w1895
          tunnel: [w1940 w1962] -> w1894
          tunnel: [w1939 w1961] -> w1893
          frame False {
          }
          frame True {
            n1701 = Tick Count (ms)() -> (millisecond timer value=w1998:u32)
            n1702 = String To Byte Array(string=w1967) -> (unsigned byte array=w2011:u8[])
            n1703 = Array Size(array=w2011) -> (size(s)=w2010:i32)
            n1704 = formula code="// --- INTERNAL VARIABLE DECLARATIONS ---\nint i = 0;\nint k = 0;\nint start_idx = -1;\nint end_idx = -1;\nint phase = 0;\nint sign0 = 1;\nint sign1 = 1;\nint ch0_val = 0;   \nint ch1_val = 0;   \nfloat ch0_raw = 0.0;\nfloat ch1_raw = 0.0;\nfloat temp0 = 0.0;\nfloat temp1 = 0.0;\nfloat ch0_clean = 0.0;\nfloat ch1_clean = 0.0;\n\nint valid_samples = 0; // FIX: Track if we actually parsed new data this window\nfloat max_allowed_bits = 8388607.0; // FIX: Change this to match your ADC max value\n\n// Temporal intermediate variables for calculation smoothing\nfloat raw_p2p_v = 0.0;\nfloat raw_friction = 0.0;\nfloat raw_cof = 0.0;\n\n// Temporal intermediate variables for Piezo voltage translations\nfloat piezo_min_v = 0.0;\nfloat piezo_max_v = 0.0;\n\n// Initialize output variables to current shift register states right away\nout_LVDT_Min_V = in_LVDT_Min_V;\nout_LVDT_Max_V = in_LVDT_Max_V;\nout_LVDT_P2P_V = in_LVDT_P2P_V;\nout_Piezo_P2P = in_Piezo_P2P;\nout_Friction_N = in_Friction_N;\nout_COF = in_COF;\nwindow_ready = 0;\n\n// --- STEP 1: PARSE EVERY STRING IN THE BYTE ARRAY ---\nif (array_size > 2) {\n    for (i = 0; i < array_size - 1; i++) {\n        if (raw_bytes[i] == 42) { // '*' character detected\n            start_idx = i;\n        }\n        \n        // Match standard delimiter sequence \";&\" or end window character\n        if (raw_bytes[i] == 59 && raw_bytes[i+1] == 38 && start_idx != -1) { \n            end_idx = i;\n            ch0_val = 0;\n            ch1_val = 0;\n            sign0 = 1;\n            sign1 = 1;\n            phase = 0; \n\n            for (k = start_idx + 1; k < end_idx; k++) {\n                if (raw_bytes[k] == 45) { // '-' sign\n                    if (phase == 0) sign0 = -1;\n                    else sign1 = -1;\n                }\n                else if (raw_bytes[k] == 43) { // '+' sign\n                    if (phase == 0) sign0 = 1;\n                    else sign1 = 1;\n                }\n                else if (raw_bytes[k] == 59) { // ';' delimiter\n                    phase = 1; \n                }\n                else if (raw_bytes[k] >= 48 && raw_bytes[k] <= 57) { // Numeric ASCII digits\n                    if (phase == 0) {\n                        ch0_val = (ch0_val * 10) + (raw_bytes[k] - 48);\n                    } else {\n                        ch1_val = (ch1_val * 10) + (raw_bytes[k] - 48);\n                    }\n                }\n            }\n\n            // Implicit type conversion\n            ch0_raw = ch0_val * sign0 * 1.0;\n            ch1_raw = ch1_val * sign1 * 1.0;\n\n            // FIX: Sanity check / Hard-clamping to catch sudden massive ASCII noise spikes\n            if (ch0_raw > max_allowed_bits)  ch0_raw = max_allowed_bits;\n            if (ch0_raw < -max_allowed_bits) ch0_raw = -max_allowed_bits;\n            if (ch1_raw > max_allowed_bits)  ch1_raw = max_allowed_bits;\n            if (ch1_raw < -max_allowed_bits) ch1_raw = -max_allowed_bits;\n\n            // --- STEP 2: 3-SAMPLE MEDIAN FILTER ---\n            m0_2 = m0_1; m0_1 = m0_0; m0_0 = ch0_raw;\n            float s0_0 = m0_0; float s0_1 = m0_1; float s0_2 = m0_2;\n            if (s0_0 > s0_1) { temp0 = s0_0; s0_0 = s0_1; s0_1 = temp0; }\n            if (s0_1 > s0_2) { temp0 = s0_1; s0_1 = s0_2; s0_2 = temp0; }\n            if (s0_0 > s0_1) { temp0 = s0_0; s0_0 = s0_1; s0_1 = temp0; }\n            ch0_clean = s0_1;\n\n            m1_2 = m1_1; m1_1 = m1_0; m1_0 = ch1_raw;\n            float s1_0 = m1_0; float s1_1 = m1_1; float s1_2 = m1_2;\n            if (s1_0 > s1_1) { temp1 = s1_0; s1_0 = s1_1; s1_1 = temp1; }\n            if (s1_1 > s1_2) { temp1 = s1_1; s1_1 = s1_2; s1_2 = temp1; }\n            if (s1_0 > s1_1) { temp1 = s1_0; s1_0 = s1_1; s1_1 = temp1; }\n            ch1_clean = s1_1;\n\n            // --- STEP 3: EXPONENTIAL FILTER (STREAM LEVEL) ---\n            if (ch0_filt == 0.0) ch0_filt = ch0_clean;\n            if (ch1_filt == 0.0) ch1_filt = ch1_clean;\n\n            ch0_filt = ch0_filt + (ch0_clean - ch0_filt) * 0.125;\n            ch1_filt = ch1_filt + (ch1_clean - ch1_filt) * 0.125;\n\n            // --- STEP 4: MIN/MAX WINDOW CONTINUOUS ACCUMULATION ---\n            if (ch0_filt > max_ch0) max_ch0 = ch0_filt;\n            if (ch0_filt < min_ch0) min_ch0 = ch0_filt;\n            if (ch1_filt > max_ch1) max_ch1 = ch1_filt;\n            if (ch1_filt < min_ch1) min_ch1 = ch1_filt;\n\n            valid_samples++; // FIX: Successfully parsed and accumulated a clean point\n            start_idx = -1; \n        }\n    }\n}\n\n// --- STEP 5: WINDOW EVALUATION ENGINE ---\n// FIX: Condition updated to verify that valid samples exist for both channels\nif (((current_time_ms - start_time_ms) >= 50) && (valid_samples > 0) && (min_ch0 < 9000000.0) && (min_ch1 < 9000000.0)) {\n    window_ready = 1;\n\n    // Linear Bit-to-Voltage Transformations (LVDT - Channel 0)\n    out_LVDT_Min_V = (min_ch0 * VREF) / 8388607.0;\n    out_LVDT_Max_V = (max_ch0 * VREF) / 8388607.0;\n    raw_p2p_v = out_LVDT_Max_V - out_LVDT_Min_V;\n\n    // Linear Bit-to-Voltage Transformations (Piezo - Channel 1)\n    piezo_min_v = (min_ch1 * VREF) / 8388607.0;\n    piezo_max_v = (max_ch1 * VREF) / 8388607.0;\n    \n    // Assign Peak-to-Peak Voltage directly to output indicator (Matches Python logic)\n    out_Piezo_P2P = piezo_max_v - piezo_min_v;\n    \n    // Force scaling calculations using Voltage delta * Newtons/Volt Factor\n    raw_friction = out_Piezo_P2P * PIEZO_CAL_FACTOR ;\n    raw_cof = raw_friction / NORMAL_FORCE;\n\n    // --- STEP 6: OUTPUT METRIC SMOOTHING (Low-Pass Filter Alpha = 0.05) ---\n    // Seed initial historical metrics if first loop iteration\n    if (hist_LVDT_P2P == 0.0) hist_LVDT_P2P = raw_p2p_v;\n    if (hist_Friction == 0.0) hist_Friction = raw_friction;\n    if (hist_COF == 0.0)      hist_COF = raw_cof;\n\n    // Apply exponential output dampening\n    hist_LVDT_P2P = hist_LVDT_P2P + (raw_p2p_v - hist_LVDT_P2P) * 0.05;\n    hist_Friction = hist_Friction + (raw_friction - hist_Friction) * 0.05; // Note: Can drop to 0.02 for more aggressive damping\n    hist_COF      = hist_COF + (raw_cof - hist_COF) * 0.05;\n\n    // Direct smoothed parameters out to UI Indicators\n    out_LVDT_P2P_V = hist_LVDT_P2P;\n    out_Friction_N = hist_Friction;\n    out_COF        = hist_COF;\n\n    // Reset tracking targets to extreme boundaries safely\n    min_ch0 = 9999999.0;\n    max_ch0 = -9999999.0;\n    min_ch1 = 9999999.0;\n    max_ch1 = -9999999.0;\n\n    valid_samples = 0; // FIX: Reset counter for next time frame\n    start_time_ms = current_time_ms;\n}"("raw_bytes"=w2011, "array_size"=w2010, "VREF"="VREF", "PIEZO_CAL_FACTOR"="PIEZO_CAL_FACTOR", "NORMAL_FORCE"="NORMAL_FORCE", "min_ch0"=w2006, "max_ch0"=w2005, "min_ch1"=w2004, "max_ch1"=w2003, "current_time_ms"=w1998, "start_time_ms"=w1997, "ch0_filt"=w1995, "ch1_filt"=w1994, "m0_0"=w1991, "m0_1"=w1990, "m0_2"=w1989, "m1_0"=w1988, "m1_1"=w1987, "m1_2"=w1986, "in_LVDT_Min_V"=w1979, "in_LVDT_Max_V"=w1972, "in_LVDT_P2P_V"=w1971, "in_Piezo_P2P"=w1970, "in_Friction_N"=w1969, "in_COF"=w1968, "hist_LVDT_P2P"=w1966, "hist_Friction"=w1965, "hist_COF"=w1964) -> ("window_ready"=→"Valid_data":dbl, "out_LVDT_Min_V"=w1978:dbl, "out_LVDT_Max_V"=w1977:dbl, "out_LVDT_P2P_V"=w1976:dbl, "out_Piezo_P2P"=w1975:dbl, "out_Friction_N"=w1974:dbl, "out_COF"=w1973:dbl, "min_ch0"=w2002:dbl, "max_ch0"=w2001:dbl, "min_ch1"=w2000:dbl, "max_ch1"=w1999:dbl, "start_time_ms"=w1996:u32, "ch0_filt"=w1993:dbl, "ch1_filt"=w1992:dbl, "m0_0"=w1985:dbl, "m0_1"=w1984:dbl, "m0_2"=w1983:dbl, "m1_0"=w1982:dbl, "m1_1"=w1981:dbl, "m1_2"=w1980:dbl, "hist_LVDT_P2P"=w1963:dbl, "hist_Friction"=w1962:dbl, "hist_COF"=w1961:dbl)
            "LVDT MIN" <- w1978
            "LVDT MAX" <- w1977
            "LVDT Peak" <- w1976
            "pizo raw" <- w1975
            "cof" <- w1973
            "Frictioin Force Raw" <- w1974
          }
        }
      }
      frame Error {
      }
    }
    n1705 = local read "Quit"() -> (w1892:bool)
  }
  n1706 = disable-structure shown="Disabled" {
    disable-tunnel: errorcluster {"status"=TRUE, "code"=0, "source"="Init"} ("error IO") -> [w2037 _]
    disable-tunnel: [w2035 _] -> w47
    frame Disabled {
      n1707 = while {
        shift-right: [w2053] -> w2039
        shift-left: _ -> [w2044]
        shift-right: [w2052] -> w2038
        shift-left: w2037 -> [w2046]
        tunnel: [w2041] -> w2035
        tunnel: [w2051] -> _
        i -> [w2051]
        stop <- w2041 stop-if-true
        n1708 = local read "Port 1a"() -> (w2047:bool)
        n1709 = local read "Port 3"() -> (w2048:bool)
        n1710 = local read "Com Port 1"() -> (w2045:refnum<visa-resource-name>)
        n1711 = Or(x=w2048, y=w2047) -> (x .or. y?=w2050:bool)
        n1712 = Unbundle(w2046) -> ("status"=→"Port 3":bool)  [unwired: 2 out]
        n1713 = Not Equal?(x=w2045, y=w2044) -> (x != y?=w2042:bool)
        n1714 = case shown="True" w2050 {
          frame False {
            w2056 = TRUE ("Visible")
            n1715 = property on="Port 1a" class="Bool (strict)"("Visible"=w2056) -> ()  [unwired: 2 in, 2 out]
            n1716 = property on="Port 3" class="Bool (strict)"("Visible"=w2056) -> ()  [unwired: 2 in, 2 out]
          }
          frame True {
            w2057 = TRUE ("Visible")
            n1717 = property on="Port 1a" class="Bool (strict)"("Visible"=w2057) -> ()  [unwired: 2 in, 2 out]
            n1718 = property on="Port 3" class="Bool (strict)"("Visible"=w2057) -> ()  [unwired: 2 in, 2 out]
          }
        }
        n1719 = Wait (ms)(milliseconds to wait=u32 40) -> ()  [unwired: 1 out]
        n1720 = case shown="True" w2042 {
          tunnel: [w2054 errorcluster {"status"=TRUE, "code"=0, "source"="Init"} ("error out")] -> w2043
          tunnel: w2046 -> [w2054 _]
          frame False {
          }
          frame True {
          }
        }
        n1721 = case shown="Error" w2043 {
          selector: w2043 -> [w2064 w2082]
          tunnel: [w2067 w2086] -> w2053
          tunnel: [w2066 w2080] -> w2052
          tunnel: w2044 -> [w2065 w2084]
          frame No Error {
            n1722 = property class="Instr"(reference=w2065, error in=w2064) -> (reference out=w2062:refnum<visa-resource-name>, error out=w2063:errorcluster, "Serial Settings:Number of Bytes at Serial Port"=w2059:u32)
            n1723 = Greater?(x=w2059, y=u32 5) -> (0:w2058:bool)
            n1724 = Not(x=w2058) -> (.not. x?=→"Port 1a":bool)
            n1725 = while {
              tunnel: [w2075] -> w2066
              tunnel: [w2074] -> w2067
              tunnel: w2063 -> [w2073]
              tunnel: w2062 -> [w2072]
              stop <- TRUE stop-if-true
              n1726 = property class="Instr" props=["Serial Settings:Number of Bytes at Serial Port"](reference=w2072, error in=w2073) -> (reference out=w2077:refnum<visa-resource-name>, error out=w2076:errorcluster)  [unwired: 1 out]
              n1727 = VISA Read(VISA resource name=w2077, byte count=u32 50, error in (no error)=w2076) -> (VISA resource name out=w2074:refnum<visa-resource-name>, read buffer=w2069:string, error out=w2075:errorcluster)  [unwired: 1 out]
              n1728 = Wait (ms)(milliseconds to wait=u32 5) -> ()  [unwired: 1 out]
            }
          }
          frame Error {
            w2092 = u16 0 items=["None", "XON/XOFF", "RTS/CTS", "XON/XOFF & RTS/CTS", "DTR/DSR", "XON/XOFF & DTR/DSR"] ("flow control (0:none)  2")
            w2090 = u16 10 items=["1.0"=10, "1.5"=15, "2.0"=20] ("stop bits 2")
            w2088 = u16 0 items=["None", "Odd", "Even", "Mark", "Space"] ("parity 2")